vi "UHR-Fleezers Control (host) - 12.7d.vi"() -> ()   [LabVIEW 2012] (continued)
        n2960 = xnode "Read/Write Control"("FPGA VI Reference In"=w4026, "error in"=w4025) -> ("FPGA VI Reference Out"=w4024:T20, "error out"=w4023:errorcluster, "APD 3 Gate Late Counter"=→"APD 3 Gate Late Counter":u8, "APD 3 Gate Relative Phase"=→"APD 3 Gate Relative Phase":i16)
      }
    }
    n2961 = Not Equal?(x=w3709, y="Calibration") -> (x != y?=w3668:bool)
    n2962 = case shown="True" w3668 {
      tunnel: w3707 -> [_ w4057]
      tunnel: w3706 -> [_ w4056]
      tunnel: w3705 -> [_ w4055]
      tunnel: w3702 -> [_ w4054]
      tunnel: w3642 -> [_ w4053]
      frame False {
      }
      frame True {
        n2963 = property on="Force" class="WFChart (strict)"("YScale.NameLbl.Text"=w4057) -> ()  [unwired: 2 in, 2 out]
        n2964 = property on="T2 X" class="DigNum (strict)"("Caption.Text"=w4055) -> ()  [unwired: 2 in, 2 out]
        n2965 = property on="T1 X" class="DigNum (strict)"("Caption.Text"=w4056) -> ()  [unwired: 2 in, 2 out]
        n2966 = property on="Mean" class="DigNum (strict)"("Caption.Text"=w4054) -> ()  [unwired: 2 in, 2 out]
        n2967 = property on="Difference" class="DigNum (strict)"("Caption.Text"=w4053) -> ()  [unwired: 2 in, 2 out]
      }
    }
    n2968 = Unbundle By Name(w3690) -> ("Y"=w3693:dbl[])
    n2969 = Unbundle By Name(w3687) -> ("Y"=w3696:dbl[])
    n2970 = Subtract(x=w3693, y=w3691) -> (x-y=w3694:dbl[])
    n2971 = Subtract(x=w3696, y=w3689) -> (x-y=w3695:dbl[])
    n2972 = Multiply(x=w3695, y="T2 alpha_x (nm/V)") -> (x*y=w3491:dbl[])
    n2973 = Multiply(x="T1 alpha_x (nm/V)", y=w3694) -> (x*y=w3492:dbl[])
    n2974 = Not(x="Trap Trig. Fl.") -> (.not. x?=w3528:bool)
    n2975 = Multiply(x=w3717, y=-1.0) -> (x*y=w3698:waveform(dbl))
    n2976 = Subtract(x=w3492, y=w3491) -> (x-y=w3686:dbl[])
    n2977 = Unbundle By Name(w3717) -> ("Y"=w3658:dbl[])
    n2978 = Unbundle By Name(w3718) -> ("Y"=w3493:dbl[])
    n2979 = Negate(x=w3686) -> (-x=w3489:dbl[])
    n2980 = Build Array(w3718, w3698) -> (→"Force":waveform(dbl)[])
    n2981 = Subtract(x=w3489, y="Offset (nm)") -> (x-y=w3656:dbl[])
    n2982 = call-poly <vilib>:"Mean.vi"("X"=w3658) -> ("mean"=w3495:dbl)  [unwired: 1 out]
    "T2 X" <- w3495
    n2983 = Negate(x=w3658) -> (-x=w3659:dbl[])
    n2984 = call-poly <vilib>:"Mean.vi"("X"=w3493) -> ("mean"=w3496:dbl)  [unwired: 1 out]
    "T1 X" <- w3496
    n2985 = Negate(x=w3495) -> (-x=w3494:dbl)
    n2986 = Bundle By Name(cluster=w3690, "Y"=w3656) -> (w3634:waveform(dbl))
    "Bead Separation" <- w3634
    n2987 = Add(x=w3493, y=w3659) -> (x+y=w3660:dbl[])
    n2988 = Add(x=w3496, y=w3494) -> (x+y=w3704:dbl)
    n2989 = Subtract(x=w3496, y=w3494) -> (x-y=→"Difference":dbl)
    n2990 = Divide(x=w3660, y=2.0) -> (x/y=→"Vec Mean of T1 T2":dbl[])
    n2991 = Divide(x=w3704, y=2.0) -> (x/y=w3662:dbl)
    "Mean" <- w3662
    n2992 = feedback-in #25("Trap Trig. Fl.") -> ()
    n2993 = feedback #25("Trap Trig. Fl.") -> (w3526:bool)
    n2994 = And(x=w3528, y=w3526) -> (x .and. y?=w3527:bool)
    n2995 = case "If have just turned off triggering" shown="True" w3527 {
      tunnel: w3509 -> [_ w3854]
      tunnel: w3508 -> [_ w3853]
      frame False {
      }
      frame True {
        w3852 = FALSE ("FPGA Trap Trig")
        n2996 = xnode "Read/Write Control"("FPGA VI Reference In"=w3854, "error in"=w3853, "FPGA Trap Trig"=w3852) -> ("FPGA VI Reference Out"=w3851:T20, "error out"=w3850:errorcluster)
        n2997 = xnode "Read/Write Control"("FPGA VI Reference In"=w3851, "error in"=w3850, "TTrig?"=w3852) -> ()  [unwired: 2 out]
        n2998 = local write "Initializing"(FALSE ("Initializing")) -> ()
        n2999 = local write "Triggered"(FALSE ("Triggered")) -> ()
        n3000 = local write "Waiting"(FALSE ("Waiting")) -> ()
      }
    }
    n3001 = Not(x=w3526) -> (.not. x?=w3539:bool)
    n3002 = And(x="Trap Trig. Fl.", y=w3539) -> (x .and. y?=w3536:bool)
    n3003 = local read "Tether"() -> (w3663:bool)
    n3004 = Or(x=w3536, y="Reinitialize") -> (x .or. y?=w3522:bool)
    n3005 = feedback #26(w3532) -> (w3537:string)
    n3006 = Select(t=w3532, s=w3536, f=w3537) -> (s? t:f=w3531:string)
    n3007 = Select(t=w3532, s="Reinitialize", f=w3531) -> (s? t:f=w3530:string)
    n3008 = feedback #27(0) -> (w3534:i32)
    n3009 = feedback #28(w3656) -> (w3655:dbl[])
    n3010 = Build Array (concatenate)(w3656, w3655) -> (w3490:dbl[])
    n3011 = case "For determining if there is a tether still" shown="True" w3663 {
      tunnel: w3662 -> [_ w3978]
      frame False {
      }
      frame True {
        n3012 = Greater?(x="Lost Tether Alarm Threshold (pN)", y=w3978) -> (0:w3976:bool)
        n3013 = case shown="True" w3976 {
          frame False {
          }
          frame True {
            w3979 = FALSE ("Value (Signaling)")
            n3014 = flat-sequence {
              frame #0 {
                # "stop only if saving"
                n3015 = local read "Saving..."() -> (w3991:bool)
                n3016 = And(x=w3991, y="TA Cancel Save?") -> (x .and. y?=w3990:bool)
                n3017 = local write "Stop Saving"(w3990) -> ()
              }
              frame #1 {
                n3018 = case shown="True" "TA Green Off?" {
                  frame False {
                  }
                  frame True {
                    w3994 = FALSE ("Fl. Triggered...")
                    n3019 = local write "Fl. Triggered..."(w3994) -> ()
                    n3020 = property on="Green Laser ON" class="Bool (strict)"("Val(Sgnl)"=w3994) -> ()  [unwired: 2 in, 2 out]
                  }
                }
              }
            }
            n3021 = local read "Time tether formed"() -> (w3985:timestamp)
            n3022 = Get Date/Time In Seconds() -> (seconds since 1Jan1904=w3986:timestamp)
            n3023 = Subtract(x=w3986, y=w3985) -> (x-y=w3984:dbl)
            n3024 = Number To Decimal String(number=w3984) -> (decimal integer string=w3981:string)  [unwired: 1 out]
            n3025 = local read "Messages"() -> (w3988:string)
            n3026 = call <vilib>:"Beep.vi"() -> ()  [unwired: 3 in, 9 out]
            n3027 = Concatenate Strings("Lost tether (" ("Message to add"), w3981, " s)." ("string")) -> (w3983:string)
            n3028 = local write "Tether"(FALSE ("Tether")) -> ()
            n3029 = call "Update messages.vi"("Message to add"=w3983, "Old message string"=w3988) -> ("New message string"=w3987:string)
            n3030 = local write "Messages"(w3987) -> ()
            n3031 = property on="Fl. Triggered..." class="Bool (strict)"("Val(Sgnl)"=w3979) -> ()  [unwired: 2 in, 2 out]
            n3032 = local write "Dip for Protein"(w3979) -> ()
            n3033 = property on="Trap Pos. FB ON" class="Bool (strict)"("Val(Sgnl)"=w3979) -> ()  [unwired: 2 in, 2 out]
            n3034 = property on="Trap Trig. Fl." class="Bool (strict)"("Val(Sgnl)"=w3979) -> ()  [unwired: 2 in, 2 out]
          }
        }
      }
    }
    n3035 = case "For triggering actions based on the trap position (e.g., turning the excitation laser on if trap under feedback moves so far)" shown="True" "Trap Trig. Fl." {
      tunnel: w3517 -> [_ w3867]
      tunnel: w3530 -> [_ w3866]
      tunnel: ["" ("t") w3865] -> w3538
      tunnel: w3522 -> [_ w3864]
      tunnel: [0 ("t") w3863] -> w3535
      tunnel: w3534 -> [_ w3862]
      tunnel: w3509 -> [_ w3861]
      tunnel: w3508 -> [_ w3860]
      frame False {
      }
      frame True {
        n3036 = case shown="\"Wait for trigger\"" w3866 {
          tunnel: w3867 -> [w3884 _ _ w3932]
          tunnel: [w3881 w3913 "" ("t") w3935] -> w3865
          tunnel: w3864 -> [_ _ _ w3923]
          tunnel: [w3880 w3910 0 ("t") w3924] -> w3863
          tunnel: w3862 -> [_ w3912 _ w3930]
          tunnel: w3861 -> [w3869 w3907 _ w3926]
          tunnel: w3860 -> [w3868 w3906 _ w3925]
          frame "Wait for trigger" {
            n3037 = local read "Trap Trig. (FPGA)"() -> (w3872:bool)
            n3038 = Subtract(x=w3884, y="Mean T1 Position\nto compare (nm)") -> (x-y=w3877:dbl[])
            n3039 = call <vilib>:"Std Deviation and Variance.vi"("X"=w3877) -> ("mean"=→"mean":dbl, "standard deviation"=→"standard\ndeviation":dbl)  [unwired: 1 in, 1 out]
            n3040 = Array Max & Min(array=w3877) -> (max value=→"max value":dbl, min value=→"min value":dbl)  [unwired: 2 out]
            n3041 = Greater?(x=w3877, y="Threshold (nm)") -> (0:w3887:bool[])
            n3042 = case shown="True" w3872 {
              tunnel: w3869 -> [_ w3893]
              tunnel: w3868 -> [_ w3892]
              tunnel: [FALSE ("TTrig?") w3891] -> w3875
              frame False {
              }
              frame True {
                n3043 = xnode "Read/Write Control"("FPGA VI Reference In"=w3893, "error in"=w3892) -> ("TTrig?"=w3891:bool)  [unwired: 2 out]
              }
            }
            n3044 = Or Array Elements(Boolean array=w3887) -> (logical OR=w3874:bool)
            n3045 = Select(t=w3875, s=w3872, f=w3874) -> (s? t:f=w3873:bool)
            n3046 = Not(x=w3872) -> (.not. x?=w3871:bool)
            n3047 = And(x=w3873, y=w3871) -> (x .and. y?=w3870:bool)
            n3048 = Select(t="Triggered", s=w3873, f="Wait for trigger") -> (s? t:f=w3881:string)
            n3049 = case shown="True" w3873 {
              tunnel: [0 0] -> w3880
              tunnel: w3869 -> [_ w3898]
              tunnel: w3868 -> [_ w3897]
              frame False {
                "Waiting" <- TRUE ("Waiting")
              }
              frame True {
                n3050 = xnode "Read/Write Control"("FPGA VI Reference In"=w3898, "error in"=w3897, "TTrig?"=FALSE) -> ()  [unwired: 2 out]
                n3051 = local read "Messages"() -> (w3901:string)
                n3052 = call <vilib>:"Beep.vi"() -> ()  [unwired: 12 in]
                n3053 = call "Update messages.vi"("Message to add"="Unwinding trigger.", "Old message string"=w3901) -> ("New message string"=w3902:string)
                n3054 = local write "Messages"(w3902) -> ()
                n3055 = local write "Waiting"(FALSE ("Waiting")) -> ()
                "Triggered" <- TRUE ("Triggered")
              }
            }
            n3056 = case "Only need to turn on laser if host triggered" shown="True" w3870 {
              frame False {
              }
              frame True {
                n3057 = property on="Green Laser ON" class="Bool (strict)"("Val(Sgnl)"=TRUE ("Value (Signaling)")) -> ()  [unwired: 2 in, 2 out]
              }
            }
          }
          frame "Triggered" {
            n3058 = local read "Trap Trig. (FPGA)"() -> (w3909:bool)
            n3059 = Increment(x=w3912) -> (x+1=w3910:i32)
            n3060 = Greater Or Equal?(x=w3910, y="Fl. ON time (n)") -> (x >= y?=w3908:bool)
            n3061 = Select(t="Wait for trigger", s=w3908, f="Triggered" ("t")) -> (s? t:f=w3913:string)
            n3062 = And(x=w3908, y=w3909) -> (x .and. y?=w3905:bool)
            n3063 = case shown="True" w3905 {
              tunnel: w3907 -> [_ w3917]
              tunnel: w3906 -> [_ w3916]
              frame False {
              }
              frame True {
                n3064 = xnode "Read/Write Control"("FPGA VI Reference In"=w3917, "error in"=w3916, "FPGA Trap Trig"=TRUE) -> ()  [unwired: 2 out]
              }
            }
            n3065 = case shown="True" w3908 {
              frame False {
              }
              frame True {
                w3919 = FALSE ("Value (Signaling)")
                n3066 = local write "Triggered"(w3919) -> ()
                n3067 = local write "Waiting"(TRUE ("Waiting")) -> ()
                n3068 = property on="Green Laser ON" class="Bool (strict)"("Val(Sgnl)"=w3919) -> ()  [unwired: 2 in, 2 out]
              }
            }
          }
          frame "Do nothing" {
          }
          frame "Initialize", Default {
            n3069 = Increment(x=w3930) -> (x+1=w3934:i32)
            n3070 = Select(t=1, s=w3923, f=w3934) -> (s? t:f=w3924:i32)
            n3071 = feedback #29(w3932) -> (w3938:dbl[])
            n3072 = Build Array (concatenate)(w3932, w3938) -> (w3931:dbl[])
            n3073 = Greater Or Equal?(x=w3924, y="Wait to get offset (n)") -> (x >= y?=w3927:bool)
            n3074 = Select(t=w3932, s=w3923, f=w3931) -> (s? t:f=w3933:dbl[])
            n3075 = feedback-in #29(w3933) -> ()
            n3076 = call-poly <vilib>:"Mean.vi"("X"=w3933) -> ("mean"=w3928:dbl)  [unwired: 1 out]
            n3077 = local write "Mean T1 Position\nto compare (nm)"(w3928) -> ()
            n3078 = case shown="True" w3923 {
              tunnel: w3926 -> [_ w3944]
              tunnel: w3925 -> [_ w3943]
              frame False {
              }
              frame True {
                w3940 = FALSE ("FPGA Trap Trig")
                n3079 = xnode "Read/Write Control"("FPGA VI Reference In"=w3944, "error in"=w3943, "FPGA Trap Trig"=w3940) -> ("FPGA VI Reference Out"=w3942:T20, "error out"=w3941:errorcluster)
                n3080 = xnode "Read/Write Control"("FPGA VI Reference In"=w3942, "error in"=w3941, "TTrig?"=w3940) -> ()  [unwired: 2 out]
              }
            }
            n3081 = Select(t="Wait for trigger", s=w3927, f="Initialize") -> (s? t:f=w3935:string)
            n3082 = case shown="True" w3927 {
              tunnel: w3928 -> [_ w3947]
              tunnel: w3926 -> [_ w3956]
              tunnel: w3925 -> [_ w3955]
              frame False {
                n3083 = local write "Waiting"(FALSE ("Waiting")) -> ()
                "Initializing" <- TRUE ("Initializing")
              }
              frame True {
                n3084 = local read "Threshold (nm)"() -> (w3959:dbl)
                n3085 = local read "AOM X Cal (nm/MHz)"() -> (w3958:dbl)
                n3086 = Add(x=w3947, y=w3959) -> (x+y=w3960:dbl)
                n3087 = Divide(x=w3960, y=w3958) -> (x/y=w3957:dbl)
                n3088 = call "IR AOM freq to word.vi"("Frequency In (MHz)"=w3957) -> ("Frequency Word Out (double)"=w3954:dbl)
                n3089 = local write "Initializing"(FALSE ("Initializing")) -> ()
                n3090 = local write "Waiting"(TRUE ("Waiting")) -> ()
                n3091 = To Quad Integer(1:w3954) -> (0:w3953:i64)
                n3092 = xnode "Read/Write Control"("FPGA VI Reference In"=w3956, "error in"=w3955, "FPGA TTrig Thresh"=w3953) -> ("FPGA VI Reference Out"=w3950:T20, "error out"=w3949:errorcluster)
                n3093 = xnode "Read/Write Control"("FPGA VI Reference In"=w3950, "error in"=w3949, "FPGA Trap Trig"=TRUE) -> ()  [unwired: 2 out]
              }
            }
          }
        }
      }
    }
    n3094 = feedback-in #26(w3538) -> ()
    n3095 = feedback-in #27(w3535) -> ()
    n3096 = Split 1D Array(array=w3490, index=w3552) -> (first subarray=w3652:dbl[])  [unwired: 1 out]
    n3097 = feedback-in #28(w3652) -> ()
    n3098 = call-poly <vilib>:"Mean.vi"("X"=w3652) -> ("mean"=w3651:dbl)  [unwired: 1 out]
    "Bead Mean (nm)" <- w3651
    n3099 = Subtract(x=w3652, y=w3651) -> (x-y=w3650:dbl[])
    n3100 = Square(x=w3650) -> (x^2=w3649:dbl[])
    n3101 = call-poly <vilib>:"Mean.vi"("X"=w3649) -> ("mean"=w3648:dbl)  [unwired: 1 out]
    n3102 = Square Root(x=w3648) -> (sqrt(x)=w3647:dbl)
    n3103 = Multiply(x=10.0, y=w3647) -> (x*y=→"RMS (Ang)":dbl)
    n3104 = xnode ("Read/Write Control")("FPGA VI Reference In"=w3684, "error in"=w3683) -> ("FPGA VI Reference Out"=w3520:T20, "error out"=w3519:errorcluster, "AI2 Y Sum Set 1"=w3781:i16, "AI2 Y Sum Set 2"=w3780:i16, "AI1 X Set 1"=w3584:fxp<+/-,16,1>, "AI1 X Set 2"=w3583:fxp<+/-,16,1>, "Trap Pos FB Int Signal"=→"Trap Pos FB Int Signal":fxp<+/-,24,9>, "Trap Pos FB Int-Norm Signal"=→"Trap Pos FB Int-Norm Signal":fxp<+/-,16,1>, "Trap Pos FB Action"=w3577:i64, "Scanning"=→"AOD Scanning":bool, "Scan I"=→"AOD Scan I":u64, "Scanning MCL"=w3783:bool, "Scan I (MCL)"=→"MCL Scan I":u64, "Green FB Sum"=w3721:i16, "Trap Pos FB Action"=w3507:i64, "TTrig Fin Thresh"=w3503:i64, "Red FB Intensity"=w3484:i16, "Blue Intensity"=w3479:i16)
    "MCL Scanning" <- w3783
    "Trap Pos FB Action" <- w3577
    n3105 = Divide(x=w3484, y=3276.7) -> (x/y=w3483:dbl)
    "Red laser intensity (V)" <- w3483
    n3106 = Divide(x=w3479, y=3276.7) -> (x/y=w3478:dbl)
    "Blue laser intensity (V)" <- w3478
    n3107 = Divide(x=w3721, y=3276.7) -> (x/y=w3482:dbl)
    "Green laser intensity (V)" <- w3482
    n3108 = local read "FB Trig Integrate"() -> (w3501:u32)
    n3109 = Divide(x=w3507, y=w3501) -> (x/y=w3500:dbl)
    "TTrig Sig (Int)" <- w3500
    n3110 = Bundle(w3482, w3483, w3478) -> (→"Fluorescence laser intensities plot":cluster{dbl, dbl, dbl})  [unwired: 1 in]
    n3111 = Divide(x=w3503, y=w3501) -> (x/y=w3498:dbl)
    "TTrig Fin Thresh (Int)" <- w3498
    n3112 = local read "AOM X Cal (nm/MHz)"() -> (w3506:dbl)
    n3113 = local read "AI2 (V)"() -> (w3782:cluster{"Set 1":dbl, "Set 2":dbl})
    n3114 = Bundle By Name(cluster=w3782, "Set 1"=w3781, "Set 2"=w3780) -> (w3778:cluster{"Set 1":dbl, "Set 2":dbl})
    n3115 = Divide(x=w3577, y=327.67) -> (x/y=→"Action (%)":dbl)
    n3116 = local read "Trap X (AI1)"() -> (w3597:T10)
    n3117 = call "IR AOM word double to freq.vi"("Frequency Word In (double)"=w3498) -> ("Frequency Out (MHz)"=w3497:dbl)
    n3118 = call "IR AOM word double to freq.vi"("Frequency Word In (double)"=w3500) -> ("Frequency Out (MHz)"=w3499:dbl)
    n3119 = Divide(x=w3778, y=3276.7) -> (x/y=w3777:cluster{"Set 1":dbl, "Set 2":dbl})
    n3120 = Multiply(x=w3499, y=w3506) -> (x*y=w3505:dbl)
    "TTrig Sig (nm)" <- w3505
    n3121 = Multiply(x=w3497, y=w3506) -> (x*y=w3504:dbl)
    "TTrig Fin Thresh (nm)" <- w3504
    n3122 = local write "AI2 (V)"(w3777) -> ()
    n3123 = Bundle(cluster=w3597, "Trap 1"=w3584, "Trap 2"=w3583) -> (→"Trap X (AI1)":T10)
    n3124 = Bundle(w3505, w3504) -> (→"TTrig":cluster{dbl, dbl})  [unwired: 1 in]
    n3125 = flat-sequence "To save data" {
      tunnel: [w4867] -> w3801
      tunnel: [w4868] -> w3800
      tunnel: w3752 -> [w4861]
      tunnel: w3525 -> [w4865]
      tunnel: ["Save Calibration"] -> w3774
      tunnel: w3771 -> [w4864]
      tunnel: [w4857] -> w3770
      tunnel: [w4854] -> w3769
      tunnel: [w4851] -> w3768
      tunnel: w3751 -> [w4853]
      tunnel: w3666 -> [w4847]
      tunnel: [w4847] -> w3665
      tunnel: ["Start Saving"] -> w3635
      tunnel: [w4841] -> w3565
      tunnel: [w4840] -> w3564
      tunnel: w3801 -> [w5115]
      tunnel: w3800 -> [w5114]
      tunnel: w3566 -> [w5113]
      tunnel: w3774 -> [w5112]
      tunnel: w3770 -> [w5110]
      tunnel: w3769 -> [w5109]
      tunnel: w3768 -> [w5108]
      tunnel: w3644 -> [w5107]
      tunnel: w3676 -> [w5106]
      tunnel: w3665 -> [w5105]
      tunnel: w3635 -> [w5104]
      tunnel: w3634 -> [w5103]
      tunnel: w3462 -> [w5102]
      tunnel: w3565 -> [w5101]
      tunnel: w3564 -> [w5100]
      tunnel: w3563 -> [w5099]
      tunnel: w3486 -> [w5098]
      frame #0 {
        n3126 = Or(x="Save N Sets", y="Start Saving") -> (x .or. y?=w4848:bool)
        n3127 = To Double Precision Float(number=w4864) -> (double precision float=w4858:dbl)
        n3128 = Build Array(w4848, "Save Calibration", w4861, w4853) -> (w4863:bool[])
        n3129 = Compound Arithmetic op=OR("Save Calibration", w4861, w4848, w4853) -> (w4866:bool)
        n3130 = Boolean Array To Number(Boolean array=w4863) -> (number=w4860:u32)
        n3131 = feedback #30(FALSE ("Save APD Data\nwith Trap Data")) -> (w4842:bool)
        n3132 = feedback #31(refnum<k0> refnum) -> (w4869:refnum<file>)
        n3133 = feedback #32(refnum<k0> refnum) -> (w4844:refnum<file>)
        n3134 = feedback #33(FALSE ("Save APD Data\nwith Trap Data")) -> (w4852:bool)
        n3135 = feedback #34(refnum<k0> refnum) -> (w4855:refnum<file>)
        n3136 = feedback #35(0) -> (w4871:i32)
        n3137 = feedback #36() -> (w4859:u32)  [unwired: 1 out]
        n3138 = case shown="True" w4866 {
          tunnel: [w4878 1] -> w4867
          tunnel: w4871 -> [w4880 _]
          tunnel: [w4879 w4911] -> w4868
          tunnel: w4869 -> [w4879 _]
          tunnel: w4865 -> [_ w4929]
          tunnel: w4858 -> [_ w4927]
          tunnel: w4860 -> [_ w4930]
          tunnel: [w4877 w4910] -> w4857
          tunnel: w4859 -> [w4877 _]
          tunnel: [w4876 w4908] -> w4854
          tunnel: w4855 -> [w4876 _]
          tunnel: [w4875 w4907] -> w4851
          tunnel: w4852 -> [w4875 _]
          tunnel: "Start Saving" -> [_ w4905]
          tunnel: w4847 -> [_ w4904]
          tunnel: [w4874 w4896] -> w4840
          tunnel: w4844 -> [w4874 _]
          tunnel: [w4873 w4895] -> w4841
          tunnel: w4842 -> [w4873 _]
          frame False {
            n3139 = Increment(x=w4880) -> (x+1=w4878:i32)
          }
          frame True {
            w4901 = FALSE ("Start Saving")
            w4906 = 9.0  # File Version
            w4913 = FALSE ("prepend array or string size? (T)")
            w4912 = T26."big-endian, network order" ("byte order (0:big-endian, network order)")
            n3140 = local read "BD 1 Frequency 1 (MHz)"() -> (w4926:dbl)
            n3141 = local read "BD 2 Frequency 1 (MHz)"() -> (w4925:dbl)
            n3142 = local read "BD 1 Frequency 2 (MHz)"() -> (w4924:dbl)
            n3143 = local read "BD 2 Frequency 2 (MHz)"() -> (w4923:dbl)
            n3144 = local read "BD 1 Frequency 3 (MHz)"() -> (w4922:dbl)
            n3145 = local read "BD 2 Frequency 3 (MHz)"() -> (w4921:dbl)
            n3146 = Array Size(array=w4904) -> (size(s)=w4903:i32)
            n3147 = To Double Precision Float(number=w4903) -> (double precision float=w4902:dbl)
            n3148 = local write "Save Calibration"(w4901) -> ()
            n3149 = local write "Start Saving"(w4901) -> ()
            n3150 = Build Array("Save APD Data\nwith Trap Data", "Save Trap Pos. Data") -> (w4898:bool[])
            n3151 = Boolean Array To Number(Boolean array=w4898) -> (number=w4897:u32)
            n3152 = Build Array(w4926, w4925, w4924, w4923, w4922, w4921) -> (w4920:dbl[])
            n3153 = case shown="1, Default" w4930 {
              tunnel: w4929 -> [w5002 w5022 w5038 w5076]
              tunnel: w4902 -> [w5007 w5029 w5058 w5095]
              tunnel: w4927 -> [w5006 w5028 w5057 w5094]
              tunnel: [w5003 w5024 w5049 w5086] -> w4918
              tunnel: [w4994 "Cal sets to save" w5039 w5077] -> w4910
              tunnel: w4920 -> [w5004 w5025 w5051 w5088]
              tunnel: "Save APD Data\nwith Trap Data" -> [w5001 _ w5035 w5074]
              tunnel: [w5001 w5016 w5035 w5074] -> w4907
              tunnel: w4906 -> [w4997 w5017 w5033 w5072]
              tunnel: w4905 -> [w4996 _ _ _]
              tunnel: [w4987 w5016 w5032 w5062] -> w4895
              tunnel: "Save Trap Pos. Data" -> [w4987 _ w5032 w5062]
              tunnel: w4897 -> [w4986 _ w5031 w5061]
              frame 1, Default {
                # "timeseries"
                n3154 = case shown="True" "Profile" {
                  tunnel: [w5010 w5014] -> w4991
                  tunnel: [w5010 w5013] -> w4990
                  tunnel: [w5010 w5012] -> w4989
                  tunnel: [w5010 w5011] -> w4988
                  frame False {
                    w5010 = 0.0 ("f")
                  }
                  frame True {
                    n3155 = local read "Current Position"() -> (w5015:cluster{dbl, dbl, dbl})
                    n3156 = local read "Y change (mm)"() -> (w5011:dbl)
                    n3157 = Unbundle(w5015) -> (w5014:dbl, w5013:dbl, w5012:dbl)
                  }
                }
                n3158 = local read "Save ave N"() -> (w5009:dbl)
                n3159 = Multiply(x=w5009, y=w5002) -> (x*y=w5008:dbl)
                n3160 = To Double Precision Float(number=w4986) -> (double precision float=w5000:dbl)
                n3161 = Build Array(w4997, w5002, w5008, w5007, w5006, 0.0 ("f")) -> (w5005:dbl[])
                n3162 = Build Array(w5000, w4991, w4990, w4989, w4988) -> (w4998:dbl[])
                n3163 = Select(t=u32 4000000000, s=w4996, f="N sets to save") -> (s? t:f=w4994:u32)
                n3164 = Build Array (concatenate)(w5005, w5004, w4998) -> (w5003:dbl[])
              }
              frame 2 {
                w5019 = 0.0 ("f")
                w5016 = FALSE ("Save APD Data\nwith Trap Data")
                # "calibration"
                n3165 = Boolean To (0,1)(Boolean=w5016) -> (0, 1=w5021:i16)
                n3166 = To Double Precision Float(number=w5021) -> (double precision float=w5020:dbl)
                n3167 = Build Array(w5020, w5019, w5019, w5019, w5019) -> (w5018:dbl[])
                n3168 = Build Array(w5017, w5022, w5022, w5029, w5028, 1.0 ("t")) -> (w5026:dbl[])
                n3169 = Build Array (concatenate)(w5026, w5025, w5018) -> (w5024:dbl[])
                "Calibrating Trap..." <- TRUE ("Calibrating...")
              }
              frame 4 {
                w5036 = 0.0 ("f")
                # "scan dir (x/y = 0/1)"
                # "cycles/step"
                # "n scans (f/b)"
                # "steps"
                # "freq. range"
                # "AOD raster scan"
                n3170 = local read "Number of F/B Scans (AOD)"() -> (w5043:u16)
                n3171 = local read "Cycles/step (AOD)"() -> (w5045:u64)
                n3172 = local read "Scan Range (MHz)"() -> (w5048:dbl)
                n3173 = local read "Scan steps (AOD)"() -> (w5047:u64)
                n3174 = local read "Scan BD"() -> (w5055:bool)
                n3175 = local read "Save ave N"() -> (w5060:dbl)
                n3176 = Boolean To (0,1)(Boolean=w5055) -> (0, 1=w5054:i16)
                n3177 = To Double Precision Float(number=w5043) -> (double precision float=w5042:dbl)
                n3178 = To Double Precision Float(number=w5047) -> (double precision float=w5046:dbl)
                n3179 = To Double Precision Float(number=w5045) -> (double precision float=w5044:dbl)
                n3180 = To Double Precision Float(number=w5054) -> (double precision float=w5053:dbl)
                n3181 = Multiply(x=w5060, y=w5038) -> (x*y=w5059:dbl)
                n3182 = To Double Precision Float(number=w5031) -> (double precision float=w5037:dbl)
                n3183 = Build Array(w5037, w5036, w5036, w5036, w5036) -> (w5034:dbl[])
                n3184 = local read "N sets should be saved"() -> (w5040:dbl)
                n3185 = Build Array(w5053, w5048, w5046, w5044, w5042) -> (w5050:dbl[])
                n3186 = Build Array(w5033, w5038, w5059, w5058, w5057, 2.0 ("t")) -> (w5052:dbl[])
                n3187 = Round Toward +Infinity(x=w5040) -> (ceil(x): smallest int >= x=w5041:dbl)
                n3188 = Build Array (concatenate)(w5052, w5051, w5034, w5050) -> (w5049:dbl[])
                n3189 = To Unsigned Long Integer(number=w5041) -> (unsigned 32bit integer=w5039:u32)
              }
              frame 8 {
                w5069 = 0.0 ("f")
                # "MCL raster scan"
                n3190 = local read "Number of scans (MCL)"() -> (w5064:u64)
                n3191 = local read "Scan lines (y)"() -> (w5063:u64)
                n3192 = local read "2D or 1D Scan"() -> (w5066:bool)
                n3193 = local read "Scan Range (V)\n(of steps)"() -> (w5085:dbl)
                n3194 = local read "Fast Scan Dir"() -> (w5092:bool)
                n3195 = local read "Cycles/step (MCL)"() -> (w5082:u64)
                n3196 = local read "Scan steps (MCL)"() -> (w5084:u64)
                n3197 = Select(t=w5063, s=w5066, f=w5064) -> (s? t:f=w5065:u64)
                n3198 = Boolean To (0,1)(Boolean=w5066) -> (0, 1=w5068:i16)
                n3199 = local read "Save ave N"() -> (w5097:dbl)
                n3200 = local read "Initial X"() -> (w5071:dbl)
                n3201 = local read "Initial Y"() -> (w5070:dbl)
                n3202 = To Double Precision Float(number=w5068) -> (double precision float=w5067:dbl)
                n3203 = Boolean To (0,1)(Boolean=w5092) -> (0, 1=w5091:i16)
                n3204 = To Double Precision Float(number=w5065) -> (double precision float=w5080:dbl)
                n3205 = To Double Precision Float(number=w5084) -> (double precision float=w5083:dbl)
                n3206 = To Double Precision Float(number=w5082) -> (double precision float=w5081:dbl)
                n3207 = To Double Precision Float(number=w5091) -> (double precision float=w5090:dbl)
                n3208 = Multiply(x=w5097, y=w5076) -> (x*y=w5096:dbl)
                n3209 = To Double Precision Float(number=w5061) -> (double precision float=w5075:dbl)
                n3210 = local read "N sets should be saved (MCL)"() -> (w5078:dbl)
                n3211 = Build Array(w5075, w5067, w5069, w5069, w5069) -> (w5073:dbl[])
                n3212 = Build Array(w5090, w5085, w5083, w5081, w5080, w5071, w5070) -> (w5087:dbl[])
                n3213 = Build Array(w5072, w5076, w5096, w5095, w5094, 3.0 ("t")) -> (w5089:dbl[])
                n3214 = Round Toward +Infinity(x=w5078) -> (ceil(x): smallest int >= x=w5079:dbl)
                n3215 = Build Array (concatenate)(w5089, w5088, w5073, w5087) -> (w5086:dbl[])
                n3216 = To Unsigned Long Integer(number=w5079) -> (unsigned 32bit integer=w5077:u32)
              }
            }
            n3217 = local read "Index"() -> (w4935:dbl)
            n3218 = call "Create new save file.vi"("Insert"="", "Ext"=".dat", "Index In"=w4935) -> ("Path Out"=w4891:path, "Index Out"=w4909:dbl)
            n3219 = local write "Save file name"(w4891) -> ()
            n3220 = local write "Index"(w4909) -> ()
            n3221 = local write "Save index"(w4909) -> ()
            n3222 = Array Size(array=w4918) -> (size(s)=w4919:i32)
            n3223 = Open/Create/Replace File(file path (use dialog)=w4891, operation (0:open)=T27."create", access (0:read/write)=enum16{"read/write", "read-only", "write-only"}."write-only") -> (refnum out=w4932:refnum<file>)  [unwired: 1 in, 4 out]
            n3224 = local write "Saving..."(TRUE ("Saving...")) -> ()
            n3225 = To Double Precision Float(number=w4919) -> (double precision float=w4917:dbl)
            n3226 = String Length(string="Comment (data description)") -> (length=w4916:i32)
            n3227 = To Double Precision Float(number=w4916) -> (double precision float=w4915:dbl)
            n3228 = Deny Access(7:w4932) -> (3:w4931:refnum<file>)  [unwired: 1 in, 2 out]
            n3229 = Build Array (concatenate)(w4917, w4918, w4915) -> (w4890:dbl[])
            n3230 = case "If fluorescence data to be saved" shown="True" w4907 {
              tunnel: w4891 -> [_ w4985]
              tunnel: [refnum<k0> refnum w4965] -> w4908
              frame False {
              }
              frame True {
                w4964 = 0.0
                n3231 = local read "APD Integration Time (s)"() -> (w4970:dbl)
                n3232 = local read "N APD Samp/step"() -> (w4963:dbl)
                n3233 = local read "Number of APDs"() -> (w4962:u8)
                n3234 = Path To String(path=w4985) -> (string=w4984:string)
                n3235 = String Length(string=w4984) -> (length=w4983:i32)
                n3236 = Subtract(x=w4983, y=4) -> (x-y=w4981:i32)
                n3237 = String Subset(string=w4984, length (rest)=w4981) -> (substring=w4980:string)  [unwired: 1 out]
                n3238 = Build Array(w4970, w4963, w4962, w4964, w4964, w4964, w4964, w4964) -> (w4967:dbl[])
                n3239 = Concatenate Strings(w4980, "_fl.dat" ("string")) -> (w4978:string)
                n3240 = Array Size(array=w4967) -> (size(s)=w4969:i32)
                n3241 = String To Path(string=w4978) -> (path=w4974:path)
                n3242 = Open/Create/Replace File(file path (use dialog)=w4974, operation (0:open)=T27."create", access (0:read/write)=enum16{"read/write", "read-only", "write-only"}."write-only") -> (refnum out=w4975:refnum<file>)  [unwired: 1 in, 4 out]
                n3243 = Deny Access(7:w4975) -> (3:w4971:refnum<file>)  [unwired: 1 in, 2 out]
                n3244 = To Double Precision Float(number=w4969) -> (double precision float=w4968:dbl)
                n3245 = Build Array (concatenate)(w4968, w4967) -> (w4966:dbl[])
                n3246 = Write to Binary File(file (use dialog)=w4971, data=w4966, 5:FALSE ("prepend array or string size? (T)"), 9:T26."big-endian, network order" ("byte order (0:big-endian, network order)")) -> (refnum out=w4965:refnum<file>)  [unwired: 1 in, 3 out]
              }
            }
            n3247 = case shown="True" w4895 {
              tunnel: w4891 -> [_ w4946]
              tunnel: [refnum<k0> refnum w4945] -> w4896
              frame False {
              }
              frame True {
                w4941 = 0.0 ("element")
                n3248 = Path To String(path=w4946) -> (string=w4960:string)
                n3249 = Build Array(w4941, w4941, w4941, w4941, w4941, w4941, w4941, w4941) -> (w4942:dbl[])
                n3250 = String Length(string=w4960) -> (length=w4959:i32)
                n3251 = Subtract(x=w4959, y=4) -> (x-y=w4957:i32)
                n3252 = Array Size(array=w4942) -> (size(s)=w4944:i32)
                n3253 = String Subset(string=w4960, length (rest)=w4957) -> (substring=w4956:string)  [unwired: 1 out]
                n3254 = To Double Precision Float(number=w4944) -> (double precision float=w4943:dbl)
                n3255 = Concatenate Strings(w4956, "_pos.dat" ("string")) -> (w4954:string)
                n3256 = Build Array (concatenate)(w4943, w4942) -> (w4940:dbl[])
                n3257 = String To Path(string=w4954) -> (path=w4950:path)
                n3258 = Open/Create/Replace File(file path (use dialog)=w4950, operation (0:open)=T27."create", access (0:read/write)=enum16{"read/write", "read-only", "write-only"}."write-only") -> (refnum out=w4951:refnum<file>)  [unwired: 1 in, 4 out]
                n3259 = Deny Access(7:w4951) -> (3:w4947:refnum<file>)  [unwired: 1 in, 2 out]
                n3260 = Write to Binary File(file (use dialog)=w4947, data=w4940, 5:FALSE ("prepend array or string size? (T)"), 9:T26."big-endian, network order" ("byte order (0:big-endian, network order)")) -> (refnum out=w4945:refnum<file>)  [unwired: 1 in, 3 out]
              }
            }
            n3261 = Write to Binary File(file (use dialog)=w4931, data=w4890, 5:w4913, 9:w4912) -> (refnum out=w4914:refnum<file>)  [unwired: 1 in, 3 out]
            n3262 = Write to Binary File(file (use dialog)=w4914, data="Comment (data description)", 5:w4913, 9:w4912) -> (refnum out=w4911:refnum<file>)  [unwired: 1 in, 3 out]
            n3263 = local read "connection reference"() -> (w4893:T17)
            n3264 = Bundle("Comment (data description)"="Comment (data description)", "Channel 1 Buffer"="Channel 1 Buffer", "Channel 2 Buffer"="Channel 2 Buffer", "Channel 3 Buffer"="Channel 3 Buffer", "Title"="Title", "DNA Construct"="DNA Construct", "Bead diameter"="Bead diameter", "Name"="Name") -> (w4881:T50)  [unwired: 1 in]
            n3265 = call "MattFileCreator-v9.vi"("Comments"=w4881, "Input Array"=w4890, "File path"=w4891, "table"="labview", "connection reference"=w4893) -> ("connection reference out"=w4892:T17)  [unwired: 5 in, 1 out]
            n3266 = local write "connection reference"(w4892) -> ()
          }
        }
        n3267 = feedback-in #30(w4841) -> ()
        n3268 = feedback-in #31(w4868) -> ()
        n3269 = feedback-in #32(w4840) -> ()
        n3270 = feedback-in #33(w4851) -> ()
        n3271 = feedback-in #34(w4854) -> ()
        n3272 = feedback-in #35(w4867) -> ()
        n3273 = feedback-in #36(w4857) -> ()
      }
      frame #1 {
        n3274 = local read "Saving..."() -> (w5111:bool)
        n3275 = case shown="True" w5111 {
          tunnel: w5115 -> [_ w5126]
          tunnel: w5114 -> [_ w5140]
          tunnel: w5113 -> [_ w5136]
          tunnel: w5112 -> [_ w5135]
          tunnel: w5110 -> [_ w5134]
          tunnel: w5109 -> [_ w5129]
          tunnel: w5108 -> [_ w5128]
          tunnel: w5107 -> [_ w5127]
          tunnel: w5106 -> [_ w5125]
          tunnel: w5105 -> [_ w5123]
          tunnel: w5104 -> [_ w5122]
          tunnel: w5103 -> [_ w5121]
          tunnel: w5102 -> [_ w5120]
          tunnel: w5101 -> [_ w5119]
          tunnel: w5100 -> [_ w5118]
          tunnel: w5099 -> [_ w5117]
          tunnel: w5098 -> [_ w5116]
          frame False {
          }
          frame True {
            n3276 = Multiply(x=w5126, y=w5125) -> (x*y=→"Time (s)":dbl)
            n3277 = Less Or Equal?(x=w5126, y=w5134) -> (x <= y?=w5138:bool)
            n3278 = Or(x="Stop Saving", y="Abort save 2") -> (x .or. y?=w5130:bool)
            n3279 = Not(x=w5130) -> (.not. x?=w5139:bool)
            n3280 = And(x=w5138, y=w5139) -> (x .and. y?=w5137:bool)
            n3281 = case shown="True" w5137 {
              tunnel: w5140 -> [w5147 w5238]
              tunnel: [0.0 w5241] -> w5133
              tunnel: w5126 -> [_ w5239]
              tunnel: w5134 -> [_ w5240]
              tunnel: w5136 -> [_ w5235]
              tunnel: w5135 -> [_ _]
              tunnel: w5129 -> [w5145 w5228]
              tunnel: w5128 -> [w5144 w5229]
              tunnel: w5127 -> [_ w5227]
              tunnel: w5123 -> [_ w5226]
              tunnel: w5122 -> [_ w5150]
              tunnel: w5121 -> [_ w5219]
              tunnel: w5120 -> [_ w5166]
              tunnel: w5119 -> [w5141 w5183]
              tunnel: w5118 -> [w5142 w5182]
              tunnel: w5117 -> [_ w5179]
              tunnel: w5116 -> [_ w5177]
              frame False {
                w5143 = FALSE
                n3282 = Close File(refnum=w5147) -> ()  [unwired: 1 in, 2 out]
                n3283 = case shown="True" w5144 {
                  tunnel: w5145 -> [_ w5149]
                  frame False {
                  }
                  frame True {
                    n3284 = Close File(refnum=w5149) -> ()  [unwired: 1 in, 2 out]
                  }
                }
                n3285 = case shown="True" w5141 {
                  tunnel: w5142 -> [_ w5148]
                  frame False {
                  }
                  frame True {
                    n3286 = Close File(refnum=w5148) -> ()  [unwired: 1 in, 2 out]
                  }
                }
                n3287 = local write "Raster Scanning..."(w5143) -> ()
                n3288 = local write "Calibrating Trap..."(w5143) -> ()
                n3289 = call <vilib>:"Beep.vi"() -> ()  [unwired: 3 in, 9 out]
                n3290 = local write "Stop Saving"(w5143) -> ()
                "Saving..." <- w5143
              }
              frame True {
                n3291 = local read "Calibrating Trap..."() -> (w5230:bool)
                n3292 = case "Write fl. data" shown="True" w5229 {
                  tunnel: w5228 -> [_ w5264]
                  tunnel: w5227 -> [_ w5263]
                  frame False {
                  }
                  frame True {
                    n3293 = Write to Binary File(file (use dialog)=w5264, data=w5263, 5:FALSE ("prepend array or string size? (T)"), 9:T26."big-endian, network order" ("byte order (0:big-endian, network order)")) -> ()  [unwired: 1 in, 4 out]
                  }
                }
                n3294 = Greater?(x="Save ave N", y=1.0) -> (0:w5233:bool)
                n3295 = Not(x=w5230) -> (.not. x?=w5232:bool)
                n3296 = And(x=w5232, y=w5233) -> (x .and. y?=w5180:bool)
                n3297 = case shown="True" w5180 {
                  tunnel: w5179 -> [w5244 w5255]
                  tunnel: [w5244 w5247] -> w5178
                  tunnel: "Save ave N" -> [_ w5248]
                  frame False {
                  }
                  frame True {
                    w5245 = 2 ("dimension size")
                    n3298 = Array Size(array=w5255) -> (size(s)=w5249:i32)
                    n3299 = Divide(x=w5249, y=w5245) -> (x/y=w5253:dbl)
                    n3300 = Reshape Array(w5255, w5253, w5245) -> (w5254:u64[][])
                    n3301 = Transpose 2D Array(2D array=w5254) -> (transposed array=w5252:u64[][])
                    n3302 = for {
                      tunnel: w5252 -> [w5257] mode=indexing
                      tunnel: [w5256] -> w5246 mode=indexing
                      tunnel: w5248 -> [w5258]
                      workers-P: _ -> [_]
                      n3303 = call "downsample 1D array - U64.vi"("Ave N"=w5258, "Array In"=w5257) -> ("Array Out"=w5256:u64[])  [unwired: 1 in]
                    }
                    n3304 = Transpose 2D Array(2D array=w5246) -> (transposed array=w5251:u64[][])
                    n3305 = Divide(x=w5249, y=w5248) -> (x/y=w5250:dbl)
                    n3306 = Reshape Array(w5251, w5250) -> (w5247:u64[])
                  }
                }
                n3307 = case shown="True" w5180 {
                  tunnel: w5235 -> [w5267 w5279]
                  tunnel: [w5267 w5271] -> w5231
                  tunnel: "Save ave N" -> [_ w5272]
                  tunnel: w5226 -> [_ w5270]
                  frame False {
                  }
                  frame True {
                    n3308 = Array Size(array=w5279) -> (size(s)=w5273:i32)
                    n3309 = Array Size(array=w5270) -> (size(s)=w5269:i32)
                    n3310 = Divide(x=w5273, y=w5269) -> (x/y=w5277:dbl)
                    n3311 = Reshape Array(w5279, w5277, w5269) -> (w5278:i16[][])
                    n3312 = Transpose 2D Array(2D array=w5278) -> (transposed array=w5276:i16[][])
                    n3313 = for {
                      tunnel: w5276 -> [w5282] mode=indexing
                      tunnel: [w5281] -> w5268 mode=indexing
                      tunnel: w5272 -> [w5280]
                      workers-P: _ -> [_]
                      n3314 = call "downsample 1D array - I16.vi"("Ave N"=w5280, "Array In"=w5282) -> ("Array Out"=w5281:i16[])  [unwired: 1 out]
                    }
                    n3315 = Transpose 2D Array(2D array=w5268) -> (transposed array=w5275:i16[][])
                    n3316 = Divide(x=w5273, y=w5272) -> (x/y=w5274:dbl)
                    n3317 = Reshape Array(w5275, w5274) -> (w5271:i16[])
                  }
                }
                n3318 = Index Array(array=w5166, index=2) -> (element=w5167:waveform(dbl))
                n3319 = Index Array(array=w5166, index=1) -> (element=w5200:waveform(dbl))
                n3320 = Index Array(array=w5166, index=0) -> (element=w5202:waveform(dbl))
                n3321 = Unbundle By Name(w5167) -> ("Y"=w5169:dbl[])
                n3322 = Unbundle By Name(w5200) -> ("Y"=w5204:dbl[])
                n3323 = Unbundle By Name(w5202) -> ("Y"=w5212:dbl[])
                n3324 = case "Write trap pos. data" shown="True" w5183 {
                  tunnel: w5182 -> [_ w5260]
                  tunnel: w5178 -> [_ w5259]
                  frame False {
                  }
                  frame True {
                    n3325 = Write to Binary File(file (use dialog)=w5260, data=w5259, 5:FALSE ("prepend array or string size? (T)"), 9:T26."big-endian, network order" ("byte order (0:big-endian, network order)")) -> ()  [unwired: 1 in, 4 out]
                  }
                }
                n3326 = Write to Binary File(file (use dialog)=w5238, data=w5231, 5:FALSE ("prepend array or string size? (T)"), 9:T26."big-endian, network order" ("byte order (0:big-endian, network order)")) -> ()  [unwired: 1 in, 4 out]
                n3327 = feedback #37(w5169) -> (w5170:dbl[])
                n3328 = Build Array (concatenate)(w5170, w5169) -> (w5165:dbl[])
                n3329 = Select(t=w5169, s=w5150, f=w5165) -> (s? t:f=w5155:dbl[])
                n3330 = feedback-in #37(w5155) -> ()
                n3331 = feedback #38(w5204) -> (w5206:dbl[])
                n3332 = Build Array (concatenate)(w5206, w5204) -> (w5205:dbl[])
                n3333 = Select(t=w5204, s=w5150, f=w5205) -> (s? t:f=w5194:dbl[])
                n3334 = feedback-in #38(w5194) -> ()
                n3335 = feedback #39(w5212) -> (w5225:dbl[])
                n3336 = Build Array (concatenate)(w5225, w5212) -> (w5224:dbl[])
                n3337 = Select(t=w5212, s=w5150, f=w5224) -> (s? t:f=w5199:dbl[])
                n3338 = feedback-in #39(w5199) -> ()
                n3339 = Divide(x=w5239, y=w5240) -> (x/y=w5242:dbl)
                n3340 = Multiply(x=w5242, y=100.0) -> (x*y=w5241:dbl)
                n3341 = Build Array(w5199, w5194, w5155) -> (→"Saved APD":dbl[][])
                n3342 = Array Size(array=w5199) -> (size(s)=w5217:i32)
                n3343 = Unbundle By Name(w5219) -> ("Y"=w5223:dbl[])
                n3344 = Subtract(x=w5217, y="N pts to average") -> (x-y=w5152:i32)
                n3345 = Multiply(x="N pts to average", y=u16 2) -> (x*y=w5195:u16)
                n3346 = Subtract(x=w5217, y=w5195) -> (x-y=w5153:i32)
                n3347 = feedback #40(w5223) -> (w5222:dbl[])
                n3348 = Build Array (concatenate)(w5222, w5223) -> (w5221:dbl[])
                n3349 = Select(t=w5223, s=w5150, f=w5221) -> (s? t:f=w5220:dbl[])
                "Trap Delta Graph" <- w5220
                n3350 = feedback-in #40(w5220) -> ()
                n3351 = Array Subset(array=w5199, index=w5152, length="N pts to average") -> (w5216:dbl[])
                n3352 = Array Subset(array=w5199, index=w5153, length="N pts to average") -> (w5215:dbl[])
                n3353 = Array Subset(array=w5194, index=w5152, length="N pts to average") -> (w5197:dbl[])
                n3354 = Array Subset(array=w5194, index=w5153, length="N pts to average") -> (w5196:dbl[])
                n3355 = Array Subset(array=w5155, index=w5152, length="N pts to average") -> (w5164:dbl[])
                n3356 = Array Subset(array=w5155, index=w5153, length="N pts to average") -> (w5163:dbl[])
                n3357 = Index Array(array=w5177, index=0) -> (element=w5175:waveform(dbl))
                n3358 = call-poly <vilib>:"Mean.vi"("X"=w5216) -> ("mean"=w5214:dbl)  [unwired: 1 out]
                n3359 = call-poly <vilib>:"Mean.vi"("X"=w5197) -> ("mean"=w5193:dbl)  [unwired: 1 out]
                n3360 = call-poly <vilib>:"Mean.vi"("X"=w5215) -> ("mean"=w5213:dbl)  [unwired: 1 out]
                n3361 = call-poly <vilib>:"Mean.vi"("X"=w5196) -> ("mean"=w5192:dbl)  [unwired: 1 out]
                n3362 = call-poly <vilib>:"Mean.vi"("X"=w5164) -> ("mean"=w5162:dbl)  [unwired: 1 out]
                n3363 = call-poly <vilib>:"Mean.vi"("X"=w5163) -> ("mean"=w5161:dbl)  [unwired: 1 out]
                n3364 = Unbundle By Name(w5175) -> ("Y"=w5173:dbl[])
                n3365 = Subtract(x=w5193, y=w5192) -> (x-y=w5184:dbl)
                "Delta Fl. 2" <- w5184
                n3366 = Subtract(x=w5162, y=w5161) -> (x-y=w5156:dbl)
                "Delta Fl. 3" <- w5156
                n3367 = Subtract(x=w5214, y=w5213) -> (x-y=w5211:dbl)
                "Delta Fl. 1" <- w5211
                n3368 = feedback #41(w5173) -> (w5172:dbl[])
                n3369 = Build Array (concatenate)(w5172, w5173) -> (w5174:dbl[])
                n3370 = Initialize Array(w5211, 1 ("dimension size")) -> (w5208:dbl[])
                n3371 = Initialize Array(w5184, 1 ("dimension size")) -> (w5189:dbl[])
                n3372 = Initialize Array(w5156, 1 ("dimension size")) -> (w5158:dbl[])
                n3373 = Select(t=w5173, s=w5150, f=w5174) -> (s? t:f=w5171:dbl[])
                "Saved trap pos" <- w5171
                n3374 = feedback-in #41(w5171) -> ()
                n3375 = feedback #42(w5208) -> (w5209:dbl[])
                n3376 = Build Array (concatenate)(w5209, w5208) -> (w5207:dbl[])
                n3377 = feedback #43(w5189) -> (w5190:dbl[])
                n3378 = feedback #44(w5158) -> (w5159:dbl[])
                n3379 = Build Array (concatenate)(w5190, w5189) -> (w5188:dbl[])
                n3380 = Build Array (concatenate)(w5159, w5158) -> (w5157:dbl[])
                n3381 = Select(t=w5208, s=w5150, f=w5207) -> (s? t:f=w5187:dbl[])
                n3382 = feedback-in #42(w5187) -> ()
                n3383 = Select(t=w5189, s=w5150, f=w5188) -> (s? t:f=w5186:dbl[])
                n3384 = feedback-in #43(w5186) -> ()
                n3385 = Select(t=w5158, s=w5150, f=w5157) -> (s? t:f=w5151:dbl[])
                n3386 = feedback-in #44(w5151) -> ()
                n3387 = Build Array(w5187, w5186, w5151) -> (→"Save APD Deriv":dbl[][])
              }
            }
            "Progress" <- w5133
            "Progress 2" <- w5133
          }
        }
      }
    }
    n3388 = local read "wait to reset values"() -> (w3785:bool)
    n3389 = Not(x=w3783) -> (.not. x?=w3786:bool)
    n3390 = And(x=w3786, y=w3785) -> (x .and. y?=w3787:bool)
    n3391 = case "Part of MCL raster scanning: returns to initial positions after scan done" shown="True" w3787 {
      tunnel: w3520 -> [w4661 w4668]
      tunnel: [w4661 w4667] -> w3789
      tunnel: w3519 -> [w4660 w4666]
      tunnel: [w4660 w4665] -> w3784
      frame False {
      }
      frame True {
        w4676 = 10.0 ("y")
        w4675 = 32767.0 ("y")
        # "to return scan values\nafter a synchronous \nAOM scan"
        n3392 = local read "AO2"() -> (w4669:dbl)
        n3393 = local read "AO1"() -> (w4670:dbl)
        n3394 = local write "wait to reset values"(FALSE ("wait to reset values")) -> ()
        n3395 = Multiply(x=w4670, y=w4675) -> (x*y=w4672:dbl)
        n3396 = Multiply(x=w4669, y=w4675) -> (x*y=w4674:dbl)
        n3397 = Divide(x=w4672, y=w4676) -> (x/y=w4671:dbl)
        n3398 = Divide(x=w4674, y=w4676) -> (x/y=w4673:dbl)
        n3399 = To Word Integer(number=w4671) -> (16bit integer=w4677:i16)
        n3400 = To Word Integer(number=w4673) -> (16bit integer=w4678:i16)
        n3401 = local read "Total Counts (ticks)"() -> (w4662:u16)
        n3402 = xnode "Read/Write Control"("FPGA VI Reference In"=w4668, "error in"=w4666, "AO1"=w4677, "AO2"=w4678, "MCL count"=w4662) -> ("FPGA VI Reference Out"=w4667:T20, "error out"=w4665:errorcluster)
        n3403 = local read "Scan Range (V)\n(of steps)"() -> (w4663:dbl)
        n3404 = property on="Scan Range (V)\n(of steps)" class="DigNum (strict)"("Val(Sgnl)"=w4663) -> ()  [unwired: 2 in, 2 out]
      }
    }
    n3405 = node-c288() -> ()  [unwired: 2 out]
  }
  n3406 = node-c288(w21) -> ()  [unwired: 1 out]
  n3407 = node-c288(w65) -> ()  [unwired: 1 out]
  n3408 = node-c288(w67) -> ()  [unwired: 1 out]
  n3409 = property on="Saved trap pos" class="WFGraph (strict)"("Visible"=FALSE) -> ()  [unwired: 2 in, 2 out]
  n3410 = property on="Trap Delta Graph" class="WFGraph (strict)"("Visible"=TRUE) -> ()  [unwired: 2 in, 2 out]
  n3411 = local write "Trap pos"(FALSE ("Trap pos")) -> ()
  n3412 = node-c288(w53) -> ()  [unwired: 1 out]
  n3413 = disable-structure shown="Disabled" {
    disable-tunnel: w57 -> [w5284 _]
    disable-tunnel: w56 -> [w5283 _]
    frame Disabled {
      n3414 = VISA Close(VISA resource name=w5284, error in (no error)=w5283) -> (error out=w5285:errorcluster)
      n3415 = call <vilib>:"Simple Error Handler.vi"("error in (no error)"=w5285) -> ()  [unwired: 1 in, 8 out]
    }
    frame Enabled {
    }
  }
  n3416 = node-c288(w63) -> ()  [unwired: 1 out]
  n3417 = node-c288(w72) -> ()  [unwired: 1 out]
  n3418 = flat-sequence {
    tunnel: w79 -> [w5289]
    tunnel: w80 -> [w5290]
    tunnel: [w5288] -> w78
    tunnel: [w5287] -> w77
    tunnel: w76 -> [_]
    tunnel: w74 -> [_]
    tunnel: w69 -> [_]
    tunnel: w78 -> [w5291]
    tunnel: w77 -> [w5292]
    frame #0 {
      w5286 = FALSE ("AI to FIFO")
      n3419 = xnode "Read/Write Control"("FPGA VI Reference In"=w5290, "error in"=w5289, "AI to FIFO"=w5286, "APD to FIFO"=w5286) -> ("FPGA VI Reference Out"=w5288:T20, "error out"=w5287:errorcluster)
    }
    frame #1 {
      n3420 = xnode "Close FPGA VI Reference"("FPGA VI Reference In"=w5291, "error in"=w5292) -> ("error out"=→"error out":errorcluster)
    }
  }
